vi "Read MFP monitor file.vi"() -> ()   [LabVIEW 2016]
uses:
  <vilib>/Utility/file.llb/Read Delimited Spreadsheet (string).vi
panel:
  in  "Tab Control":enum32{"Full graph", "Fraction of graph"}(tab)
  out "2T-G":cluster{dbl[], dbl[]}[](graph)
  out "4T-G":cluster{dbl[], dbl[]}[](graph)
  in  "Cluster":cluster{"Initial X":dbl, "Final X":dbl}
  out "4T-G 3":cluster{dbl[], dbl[]}[](graph)=[{[0.0], [nan]}]
  out "2T-G 2":cluster{dbl[], dbl[]}[](graph)
  in  "Channel settings":T1={"Drain"=11, "V+"=5, "V-"=7, "Sourcing amp (V)"=0.1, "Time (X)"=0, "Shunt resistor"=100000.0}
  out "Index, Wavenames":string[][](table)=[["0", "time"], ["1", "temp"], ["2", "humidity"], ["3", "X0"], ["4", "Y0"], ["5", "X1"], ["6", "Y1"], ["7", "X2"], ["8", "Y2"], ["9", "X3"], ["10", "Y3"], ["11", "X4"], ["12", "Y4"], ["13", "X5"], ["14", "Y5"], ["15", "X6"], ["16", "Y6"], ["17", "X7"], ["18", "Y7"]]
  out "size(s) of data":i32[](array[numeric])=[49945, 19]
  out "All Data":string[][](array[string])
  in  "Path":path=path "G:/My Drive/ansom/Data/MFP3D/Users/Yang Hu/AFM/M_3_5 N_0 (SA40161)/2020-01-19 SA40161J/Writing test/SA40161J.000000.dat"
  # "This part gets the section with X ranging from Initial X to Final X."
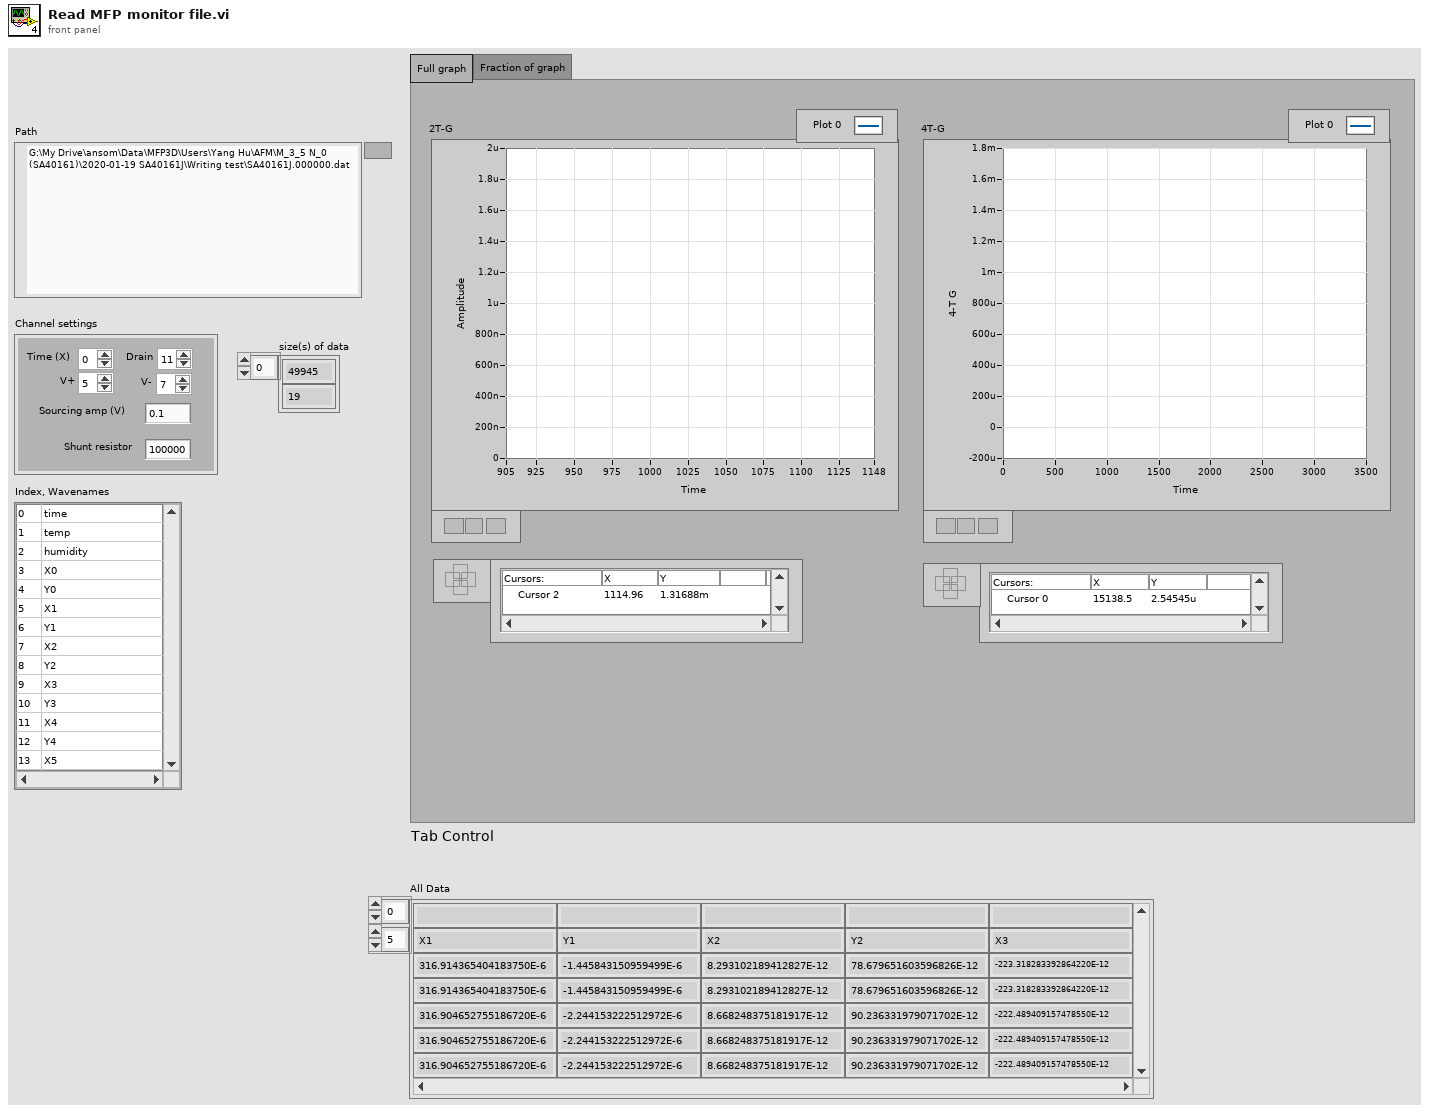
[diagram p1: front panel]
types:
  T1 = cluster{"Drain":i32, "V+":i32, "V-":i32, "Sourcing amp (V)":dbl, "Time (X)":i32, "Shunt resistor":dbl}
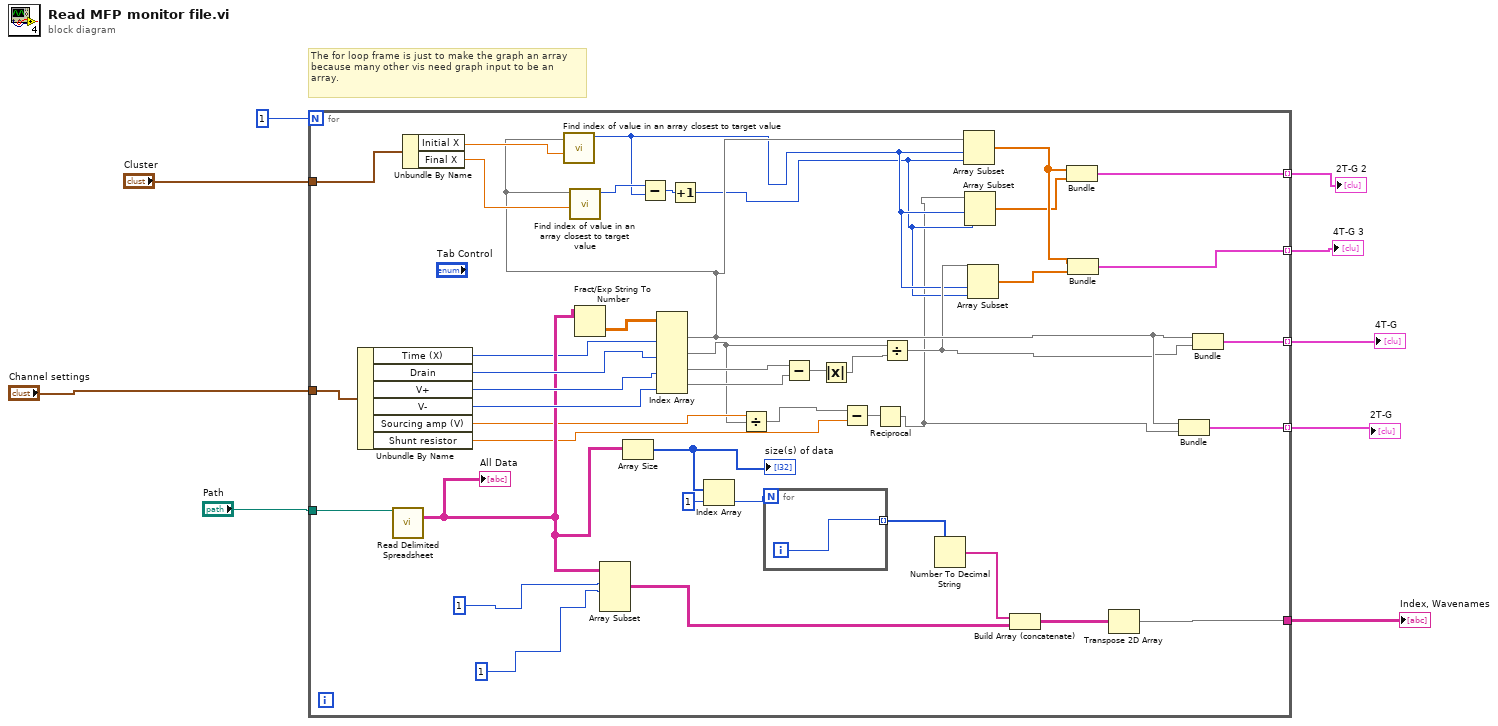
[diagram p0: block diagram]
diagram:
  # "The for loop frame is just to make the graph an array because many other vis need graph input to be an array."
  n1 = for {
    N: 1 -> [_]
    tunnel: "Path" -> [w53]
    tunnel: [w47] -> w8
    tunnel: "Channel settings" -> [w46]
    tunnel: [w41] -> w6 mode=indexing
    tunnel: [w40] -> w5 mode=indexing
    tunnel: "Cluster" -> [w29]
    tunnel: [w19] -> w2 mode=indexing
    tunnel: [w18] -> w1 mode=indexing
    n2 = Unbundle By Name(w46) -> ("Time (X)"=w31:i32, "Drain"=w39:i32, "V+"=w38:i32, "V-"=w37:i32, "Sourcing amp (V)"=w15:dbl, "Shunt resistor"=w12:dbl)
    n3 = call-poly <vilib>:"Read Delimited Spreadsheet.vi"("file path (dialog if empty)"=w53) -> ("all rows"=w36:string[][])  [unwired: 9 in, 5 out]
    "All Data" <- w36
    n4 = Unbundle By Name(w29) -> ("Initial X"=w28:dbl, "Final X"=w27:dbl)
    n5 = Fract/Exp String To Number(string=w36) -> (number=w45:dbl[][])  [unwired: 3 in, 1 out]
    n6 = Array Subset(array=w36, index (row)=1 ("index of column"), length (row)=1 ("length")) -> (w34:string[][])  [unwired: 2 in]
    n7 = Array Size(array=w36) -> (size(s)=w52:i32[])
    "size(s) of data" <- w52
    n8 = Index Array(array=w45, index (col) #1=w31, index (col) #2=w39, index (col) #3=w38, index (col) #4=w37) -> (element #1=w26:dbl[], element #2=w14:dbl[], element #3=w43:dbl[], element #4=w30:dbl[])  [unwired: 4 in]
    n9 = call "Find index of value in an array closest to target value.vi"("Target value"=w28, "Array"=w26) -> ("Index of closest value"=w22:i32)  [unwired: 8 in, 1 out]
    n10 = call "Find index of value in an array closest to target value.vi"("Target value"=w27, "Array"=w26) -> ("Index of closest value"=w25:i32)  [unwired: 8 in, 1 out]
    n11 = Subtract(x=w25, y=w22) -> (x-y=w24:i32)
    n12 = Increment(x=w24) -> (x+1=w21:i32)
    n13 = Index Array(array=w52, index=1) -> (element=w51:i32)
    n14 = Divide(x=w15, y=w14) -> (x/y=w13:dbl[])
    n15 = for {
      N: w51 -> [_]
      tunnel: [w54] -> w50 mode=indexing
      i -> [w54]
    }
    n16 = Subtract(x=w43, y=w30) -> (x-y=w44:dbl[])
    n17 = Absolute Value(x=w44) -> (abs(x)=w42:dbl[])
    n18 = Subtract(x=w13, y=w12) -> (x-y=w11:dbl[])
    n19 = Reciprocal(x=w11) -> (1/x=w10:dbl[])
    n20 = Divide(x=w14, y=w42) -> (x/y=w23:dbl[])
    n21 = Number To Decimal String(number=w50) -> (decimal integer string=w49:string[])  [unwired: 1 in]
    n22 = Array Subset(array=w26, index=w22, length=w21) -> (w17:dbl[])
    n23 = Array Subset(array=w10, index=w22, length=w21) -> (w16:dbl[])
    n24 = Array Subset(array=w23, index=w22, length=w21) -> (w20:dbl[])
    n25 = Build Array (concatenate)(w49, w34) -> (w48:string[][])
    n26 = Bundle(w17, w16) -> (w19:cluster{dbl[], dbl[]})  [unwired: 1 in]
    n27 = Bundle(w17, w20) -> (w18:cluster{dbl[], dbl[]})  [unwired: 1 in]
    n28 = Transpose 2D Array(2D array=w48) -> (transposed array=w47:string[][])
    n29 = Bundle(w26, w10) -> (w40:cluster{dbl[], dbl[]})  [unwired: 1 in]
    n30 = Bundle(w26, w23) -> (w41:cluster{dbl[], dbl[]})  [unwired: 1 in]
  }
  "Index, Wavenames" <- w8
  "4T-G" <- w6
  "2T-G" <- w5
  "2T-G 2" <- w2
  "4T-G 3" <- w1
